vi "setup_rt.vi"(6 "error in":errorcluster, 9 "Light enables":bool[](array[boolean])) -> (0 "error out":errorcluster, 2 "Micron config":T1, 3 "ASAP Config":T4)   [LabVIEW 2014]
uses:
  configuration.ctl
  asap_calibration.ctl
  <vilib>/Analysis/Matrix/Datatypes/RealMatrix.ctl
  micron/labview/initialization/micron_config.ctl
  micron/labview/manipulator/squiggle/Host/i2c_interface.ctl
  micron/labview/manipulator/squiggle/Host/fpga_reference.ctl
  micron/labview/testing/Micron params.ctl
  micron/labview/testing/stimulus.ctl
  micron/labview/testing/injection_point.ctl
  micron/labview/filtering/goal_loop_parms.ctl
  micron/labview/testing/mode_conrols.ctl
  micron/labview/testing/manipulator_cal.ctl
  testing/probe_calibration.ctl
  micron/labview/host/network_params.ctl
  micron/labview/cancellation/sq_control_params.ctl
  micron/labview/cancellation/decoupled_gain.ctl
  micron/labview/cancellation/estimation_controls.ctl
  geometry/lut4d.ctl
  globals.vi
  micron/labview/initialization/micron_globals.vi
  <vilib>/Analysis/Matrix/NI_Matrix.lvlib
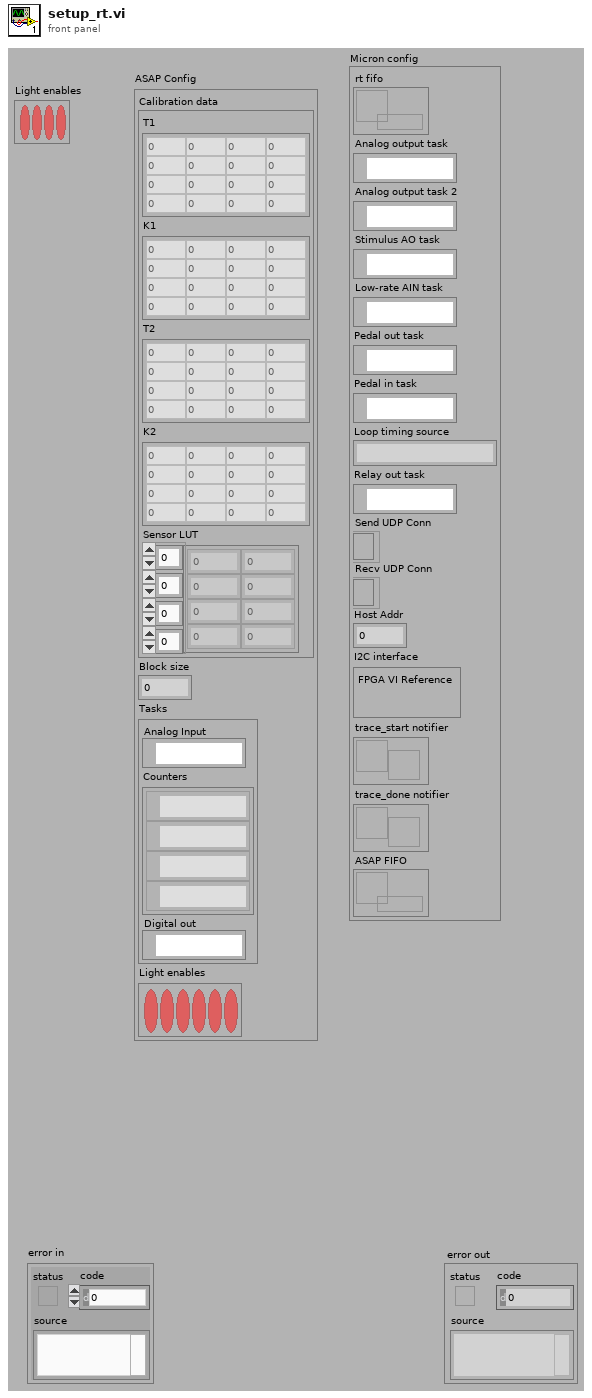
[diagram p1: front panel]
types:
  T1 = typedef "micron_config.ctl" = cluster{"rt fifo":refnum<k33>, "Analog output task":refnum<k21>, "Analog output task 2":refnum<k21>, "Stimulus AO task":refnum<k21>, "Low-rate AIN task":refnum<k21>, "Pedal out task":refnum<k21>, "Pedal in task":refnum<k21>, "Loop timing source":string, "Relay out task":refnum<k21>, "Send UDP Conn":refnum<k16>, "Recv UDP Conn":refnum<k16>, "Host Addr":u32, "I2C interface":T2, "trace_start notifier":refnum<notifier>, "trace_done notifier":refnum<notifier>, "ASAP FIFO":refnum<k33>}
  T2 = typedef "i2c_interface.ctl" = cluster{"FPGA VI Reference":T3}
  T3 = typedef "fpga_reference.ctl" = refnum<k20>
  T4 = typedef "configuration.ctl" = cluster{"Calibration data":T5, "Block size":i32, "Tasks":cluster{"Analog Input":refnum<k21>, "Counters":refnum<k21>[], "Digital out":refnum<k21>}, "Light enables":bool[]}
  T5 = typedef "asap_calibration.ctl" = cluster{"T1":T6, "K1":T6, "T2":T6, "K2":T6, "Sensor LUT":sgl[][][][]}
  T6 = typedef "NI_Matrix.lvlib/RealMatrix.ctl" = dbl[][]
  T7 = typedef "lut4d.ctl" = cluster{"Table":sgl[][][][][], "Scale":sgl[], "Offset":sgl[]}
  T8 = cluster{"Analog Input":refnum<k21>, "Counters":refnum<k21>[], "Digital out":refnum<k21>}
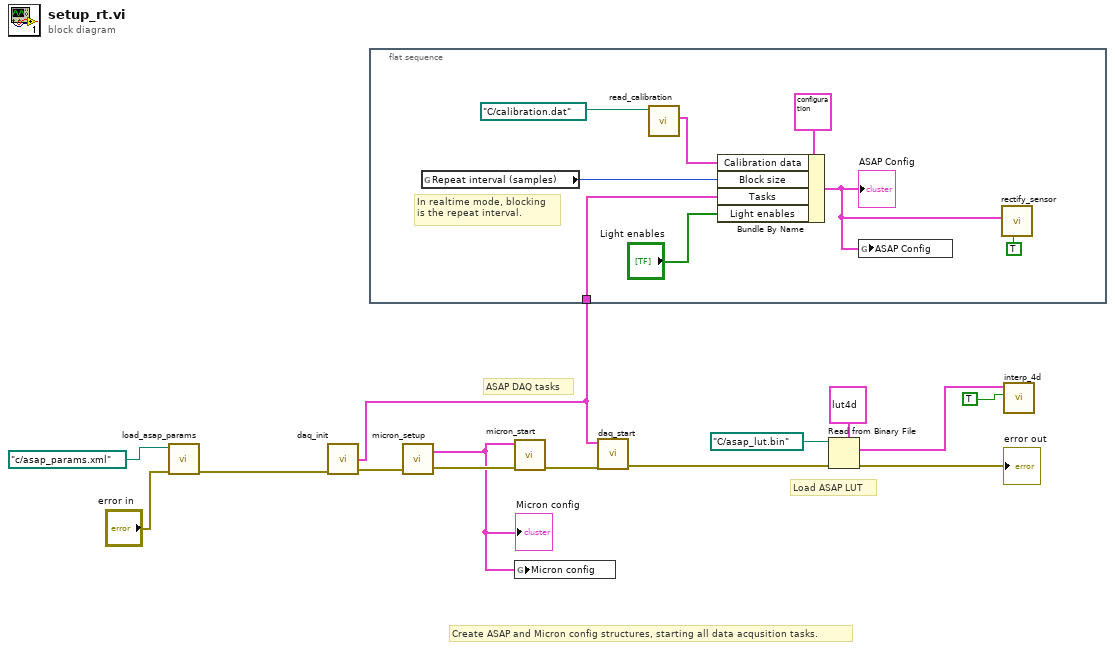
[diagram p0: block diagram]
diagram:
  # "ASAP DAQ tasks"
  # "Load ASAP LUT"
  # "Create ASAP and Micron config structures, starting all data acqusition tasks."
  n1 = call "load_asap_params.vi"("error in"="error in", "ASAP params file"=path "c:/asap_params.xml") -> ("error out"=w12:errorcluster)  [unwired: 9 out]
  n2 = call "daq_init.vi"("error in"=w12) -> ("error out"=w11:errorcluster, "Tasks"=w2:T8)  [unwired: 4 out]
  n3 = flat-sequence {
    tunnel: w2 -> [w17]
    frame #0 {
      # "In realtime mode, blocking\nis the repeat interval."
      n4 = global read "globals.vi" "Repeat interval (samples)"() -> (w18:i32)
      n5 = call "read_calibration.vi"("Calibration file name"=path "C:/calibration.dat") -> ("Calibration data"=w20:T5)  [unwired: 1 in, 9 out]
      n6 = Bundle By Name(cluster=T4 {"Calibration data"={"T1"=[], "K1"=[], "T2"=[], "K2"=[], "Sensor LUT"=[]}, "Block size"=0, "Tasks"={"Analog Input"="", "Counters"=[], "Digital out"=""}, "Light enables"=[]} ("Configuration 2"), "Calibration data"=w20, "Block size"=w18, "Tasks"=w17, "Light enables"="Light enables") -> (w16:T4)
      "ASAP Config" <- w16
      n7 = global write "micron_globals.vi" "ASAP Config"(w16) -> ()
      n8 = call "rectify_sensor.vi"("Reset"=TRUE, "Configuration"=w16) -> ()  [unwired: 9 in, 1 out]
    }
  }
  n9 = call "micron_setup.vi"("Error in"=w11) -> ("Error out"=w10:errorcluster, "Micron config"=w1:T1)  [unwired: 3 out]
  "Micron config" <- w1
  n10 = call "micron_start.vi"("error in"=w10, "Micron config"=w1) -> ("error out"=w9:errorcluster)  [unwired: 9 out]
  n11 = global write "micron_globals.vi" "Micron config"(w1) -> ()
  n12 = call "daq_start.vi"("error in"=w9, "Tasks"=w2) -> ("error out"=w4:errorcluster)  [unwired: 9 out]
  n13 = Read from Binary File(5:T7 {"Table"=array41x41x41x5x4[1378420 elements], "Scale"=[2.0, 2.0, 2.0, 0.2], "Offset"=[-1.0, -1.0, -1.0, 0.0]} ("LUT"), 8:w4, 11:path "C:/asap_lut.bin" ("Calibration file name")) -> (0:→"error out":errorcluster, 2:w5:T7)  [unwired: 5 out]
  n14 = call "interp_4d.vi"("Set LUT"=TRUE, "LUT"=w5) -> ()  [unwired: 1 in, 9 out]
